vi "Main.vi"() -> ()   [LabVIEW 2020]
uses:
  System.Windows.Forms
  Global_Variable/Global.vi
  Global_Variable/A180648.vi
  <userlib>/_MGI/Menu Building/MenuTypes/MenuStrip/MGI_MenuStrip.lvclass
  <userlib>/_MGI/Menu Building/MenuItemStatusChange/MGI_MenuItemStatusChange.lvclass
  Libraries/S7/S7.lvlib
panel:
  in  "表格控件":string[][](table)
  out "上学状态":string
  in  "Andon":enum32{"未选择", "缺料报警", "质量报警", "故障报警"}(radio)
  out "PLC":bool
  in  "菜单":refnum<k24>(container)
  out "逆向空载":bool
  out "试验计时":u16
  out "产品编号":string
  out "生产数量":i32
  out "合格数量":i32
  out "userStatus":string caption="用户状态"
  out "userName":string caption="用户名"
  out "connectionMode":string caption="联机类型"
  out "产品型号":string
  out "手柄开启力":bool
  out "手柄锁紧力":bool=TRUE
  out "振动NVH":bool
  out "备用试验1":bool
  out "备用试验2":bool
  out "手柄保持力":bool=TRUE caption="管柱保持力"
  out "锁紧/开启":bool
  out "手柄推拉力":bool caption="角度调节力"
  in  "更换产品":refnum<vi>
  out "提示信息":string
  out "错误":bool
  out "时间字符串":string
  out "日期字符串":string
  out "自动":bool
  # "手柄调节机构"
  # "试验项目"
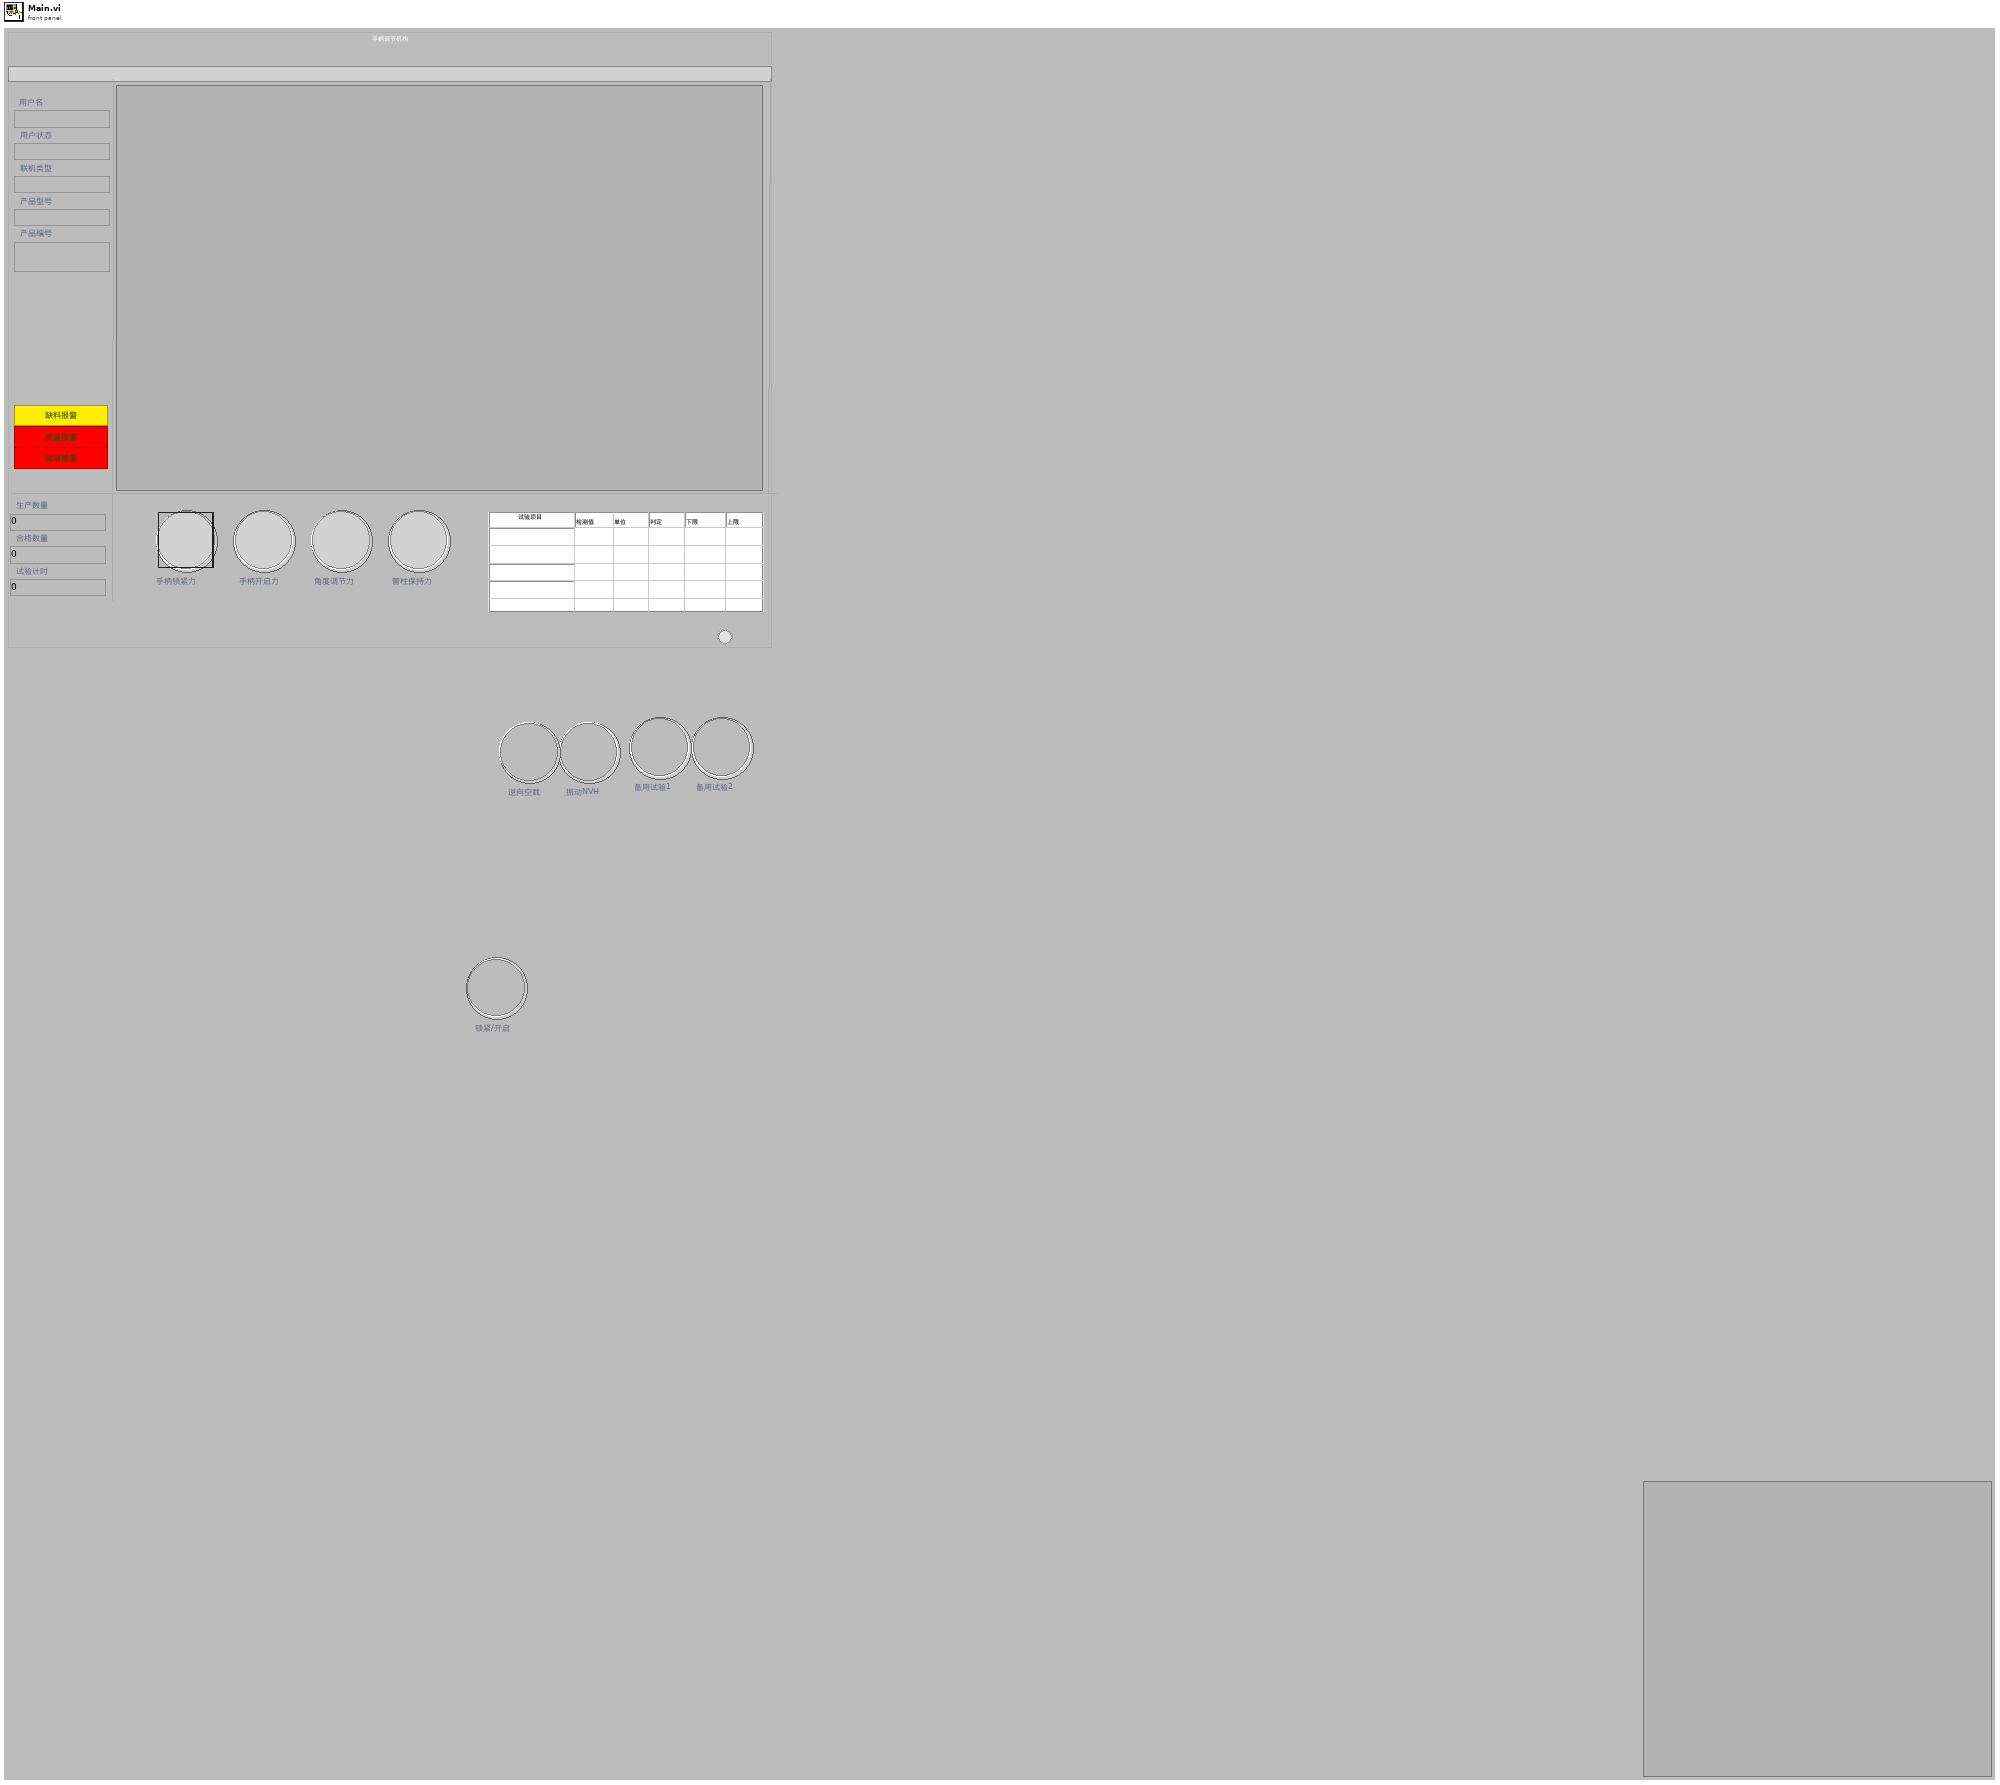
[diagram p1: front panel]
types:
  T1 = typedef "S7.lvlib/Broadcast Events--cluster.ctl" = cluster{"Module Did Init":refnum<user-event>, "Status Updated":refnum<user-event>, "Error Reported":refnum<user-event>, "Module Did Stop":refnum<user-event>, "Update Module Execution Status":refnum<user-event>}
  T2 = enum32{"手柄锁紧力", "手柄开启力", "手柄推拉力", "手柄保持力", "锁紧/松开", "逆向空载", "振动NVH"}
  T3 = enum32{"手柄锁紧力", "手柄开启力", "手柄推拉力", "手柄保持力", "锁紧/开启", "逆向空载", "振动NVH"}
  T4 = enum32{"空载", "功能", "力特性", "电流特性", "传感器特性", "逆向空载", "振动NVH"}
  T5 = enum32{"Invalid", "Standard", "Closed", "Hidden", "Minimized", "Maximized"}
  T6 = cluster{"设备名称":string, "操作人员":string, "设备状态":enum16{"设备离线", "设备正常", "设备缺料", "设备故障", "质量报警"}, "附加信息":string}
  T7 = enum32{"invalid app kind", "Development System", "Run Time System", "Student Edition", "Embedded LabVIEW", "Evaluation", "Custom"}
  T8 = cluster{"操作员编号":string, "操作员姓名":string, "操作员权限":string, "联机模式":enum16{"单机", "追溯"}}
  T9 = cluster{"Core":cluster{"Current VI Reference":refnum<vi>, "Close Panel on Exit?":bool}, "Your Boolean data":bool, "Your string data":string}
  T10 = cluster{"Current VI Reference":refnum<vi>, "Close Panel on Exit?":bool}
  T11 = cluster{"用户编号":string, "用户名":string, "用户密码(密文)":string, "用户权限":string}
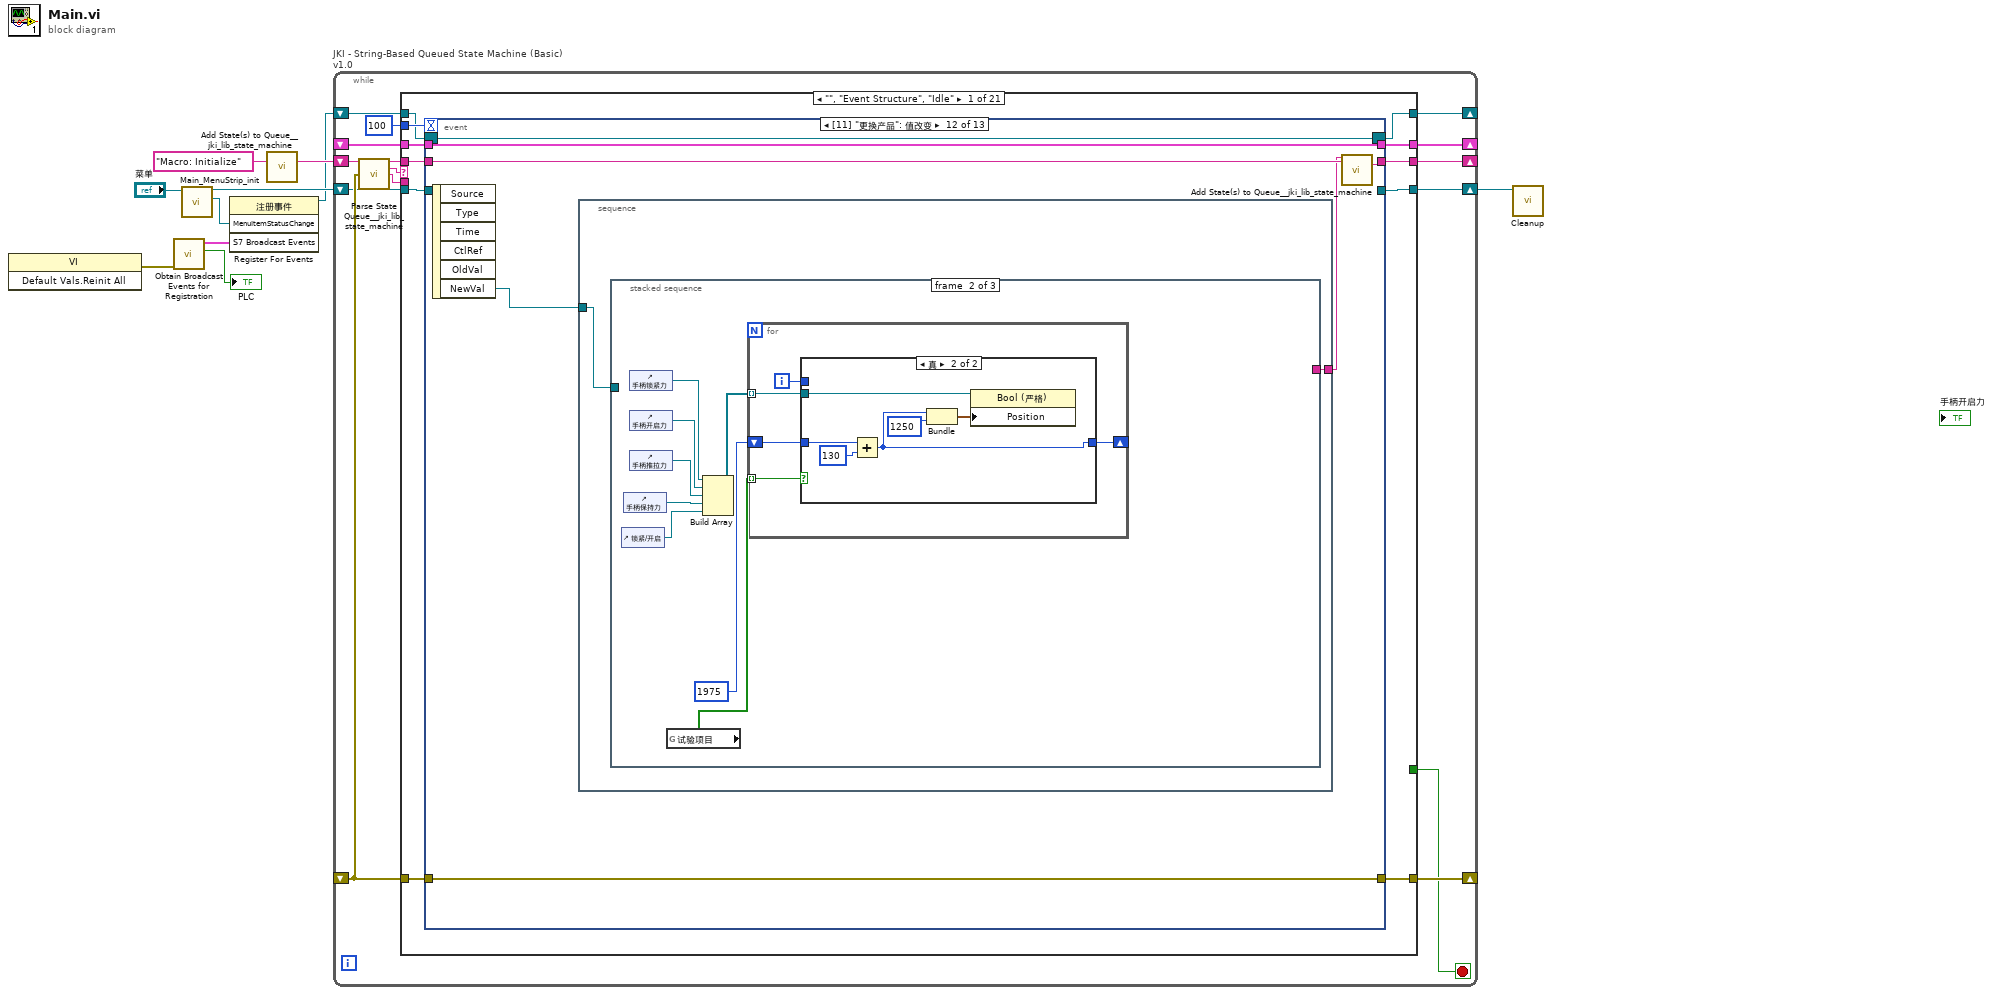
[diagram p0: block diagram]
diagram:
  n1 = invoke class="VI" method="Default Vals.Reinit All"() -> (error out=w3:errorcluster)  [unwired: 3 in, 2 out]
  n2 = call "Obtain Broadcast Events for Registration.vi"("error in (no error)"=w3) -> ("Already running?"=→"PLC":bool, "S7 Broadcast Events"=w5:T1)  [unwired: 8 in, 1 out]
  n3 = call "Main_MenuStrip_init.vi"("MenuStrip"="菜单") -> ("MenuItemStatusChange"=w2:refnum<user-event>, "Menu out"=w7:refnum<class "MGI_MenuStrip.lvclass">)  [unwired: 9 in]
  n4 = register-events(w2, w5) -> (reference out=w1:refnum<event-registration>)  [unwired: 2 in, 1 out]
  n5 = call <vilib>:"Add State(s) to Queue__jki_lib_state_machine.vi"("State(s) in (\"\")"="Macro: Initialize") -> ("States Out"=w10:string)  [unwired: 14 in]
  n6 = while "JKI - String-Based Queued State Machine (Basic) v1.0" {
    shift-right: [w19] -> _
    shift-left: _ -> [w18]
    shift-right: [w21] -> _
    shift-left: _ -> [w16]
    shift-right: [w20] -> _
    shift-left: w10 -> [w22]
    shift-right: [w14] -> w6
    shift-left: w7 -> [w15]
    shift-right: [w12] -> _
    shift-left: w1 -> [w11]
    stop <- w13 stop-if-true
    n7 = call <vilib>:"Parse State Queue__jki_lib_state_machine.vi"("State Queue"=w22, "Error In (no error)"=w16) -> ("Remaining States"=w24:string, "Current State"=w25:string, "Arguments"=w23:string)  [unwired: 11 in]
    n8 = case shown="\"\", \"Event Structure\", \"Idle\"" w25 {
      selector: w25 -> [_ _ w278 _ _ _ _ _ _ _ _ _ _ _ _ _ _ _ _ _ _]
      tunnel: w24 -> [w36 w275 w282 w302 w310 w318 w324 w328 w334 w343 w355 w363 w369 w379 w403 w443 w451 w464 w492 w499 w511]
      tunnel: w23 -> [_ _ _ _ _ _ _ _ _ _ _ _ _ _ _ _ w446 w458 _ _ _]
      tunnel: w18 -> [w34 w272 w280 w293 w307 w316 w321 w329 w337 w340 _ w358 w366 w377 w401 w440 w449 w460 w489 w496 w508]
      tunnel: [w33 w273 w284 w299 errorcluster {"status"=FALSE, "code"=0, "source"=""} ("error out") w315 w322 w326 w332 w341 w352 w359 w367 w376 w399 w441 w447 w461 w490 w497 w509] -> w21
      tunnel: w16 -> [w32 w273 w283 w299 w306 w315 w322 w326 w333 w341 w352 w360 w367 w373 w399 w441 w448 w462 w490 w497 w509]
      tunnel: [w35 w274 w281 w301 w309 w317 w323 w328 w335 w342 w354 w362 w368 w378 w402 w442 w450 w463 w491 w498 w510] -> w20
      tunnel: [w31 w272 w280 w300 w307 w316 w321 w329 w337 w340 w353 w358 w366 w377 w401 w440 w449 w460 w489 w496 w508] -> w19
      tunnel: 100 ("Timeout") -> [w30 _ _ _ _ _ _ _ _ _ _ _ _ _ _ _ _ _ _ _ _]
      tunnel: w15 -> [w29 w271 w277 w290 w304 w314 w320 w327 w336 w339 w346 w357 w365 w375 w400 w439 w445 w457 w488 w494 w501]
      tunnel: [w28 w271 w277 w290 w304 w314 w320 w327 w336 w339 w346 w357 w365 w375 w400 w439 w445 w457 w488 w494 w501] -> w14
      tunnel: [_ _ _ _ _ TRUE _ _ _ _ _ _ _ _ _ _ _ _ _ _ _] -> w13
      tunnel: [w26 w270 w276 w289 w303 w312 w319 w330 w331 w338 w347 w356 w364 w374 w398 w436 w444 w456 w487 w493 w500] -> w12
      tunnel: w11 -> [w27 w270 w276 w289 w303 w312 w319 w330 w331 w338 w347 w356 w364 w374 w398 w436 w444 w456 w487 w493 w500]
      frame "", "Event Structure", "Idle" {
        n9 = event shown="[11] \"更换产品\": 值改变" {
          selector: w27 -> [w38 w63 w84 w90 w156 w163 w170 w177 w191 w200 w207 w216 _]
          dyn-events: [w38 w63 w83 w90 w156 w163 w170 w177 w191 w200 w207 w216 _] -> w26
          timeout: w30 -> [_ _ _ _ _ _ _ _ _ _ _ _ _]
          tunnel: w36 -> [w50 w66 w88 w99 w157 w164 w173 w180 w188 w204 w214 w218 w264]
          tunnel: [w49 w65 w88 w97 w158 w165 w174 w181 w189 w205 w213 w219 w264] -> w35
          tunnel: w34 -> [w48 w67 w89 w98 w160 w168 w175 w182 w190 w206 w211 w221 w265]
          tunnel: [w39 w64 w85 w100 w161 w166 w171 w183 w186 w203 w212 w220 w262] -> w33
          tunnel: w32 -> [w39 w64 w86 w100 w161 w166 w171 w184 w186 w203 w212 w220 w262]
          tunnel: [w48 w67 w89 w98 w160 w168 w175 w182 w190 w206 w211 w221 w265] -> w31
          tunnel: w29 -> [w37 _ w87 w93 w159 w167 w172 w179 w187 _ _ _ w263]
          tunnel: [w37 _ w87 w93 w159 w167 w172 w179 w187 _ _ _ w263] -> w28
          event Timeout {
            n10 = event-data() -> ()  [unwired: 1 in, 1 out]
            n11 = global read "Global.vi" "计时开始"() -> (w41:bool)
            n12 = case shown="真" w41 {
              frame False {
                n13 = global write "Global.vi" "计时复位"(TRUE ("计时复位")) -> ()
              }
              frame True {
                n14 = stacked-sequence {
                  frame #0 {
                    n15 = global read "Global.vi" "计时复位"() -> (w52:bool)
                    n16 = call "已用时间"("Reset"=w52) -> ("Elapsed Time (s)"=→"试验计时":dbl)  [unwired: 11 in, 7 out]
                  }
                  frame #1 {
                    n17 = global write "Global.vi" "计时复位"(FALSE ("计时复位")) -> ()
                  }
                }
              }
            }
            n18 = Format Date/Time String(time format string (%c)="%H:%M ") -> (date/time string=→"时间字符串":string)  [unwired: 2 in]
            n19 = Format Date/Time String(time format string (%c)="%Y年%m月%d日") -> (date/time string=→"日期字符串":string)  [unwired: 2 in]
            n20 = call <vilib>:"Add State(s) to Queue__jki_lib_state_machine.vi"("State(s) in (\"\")"=w50) -> ("States Out"=w49:string)  [unwired: 14 in]
            n21 = global read "Global.vi" "合格数量"() -> (→"合格数量":i32)
            n22 = global read "Global.vi" "生产数量"() -> (→"生产数量":i32)
            n23 = global read "Global.vi" "产品编号"() -> (→"产品编号":string)
          }
          event "手柄锁紧力", "手柄开启力", "手柄推拉力", "手柄保持力", "锁紧/开启", "振动NVH", "逆向空载": Mouse Down {
            w55 = refnum<user-event> refnum items=["手柄锁紧力", "手柄开启力", "手柄推拉力", "手柄保持力", "锁紧/开启", "逆向空载", "振动NVH"] ("试验项_Event")
            n24 = event-data() -> ("CtlRef"=w59:refnum<vi>)  [unwired: 1 in]
            n25 = property class="Bool (严格)"(reference=w59) -> ("Label.Text"=w58:string)  [unwired: 1 in, 2 out]
            n26 = vi-ref "Auto.vi"() -> (w61:refnum<vi>)
            n27 = case shown="\"锁紧/开启\"" w58 {
              tunnel: [T2."手柄锁紧力" ("事件数据") T2."手柄开启力" ("事件数据") T2."手柄推拉力" ("事件数据") T2."手柄保持力" ("事件数据") T3."锁紧/开启" ("事件数据") T4."逆向空载" ("事件数据") T4."振动NVH" ("事件数据")] -> w56
              frame "手柄锁紧力", Default {
              }
              frame "手柄开启力" {
              }
              frame "手柄推拉力" {
              }
              frame "手柄保持力" {
              }
              frame "锁紧/开启" {
              }
              frame "逆向空载" {
              }
              frame "振动NVH" {
              }
            }
            n28 = invoke class="VI" method="Ctrl Val.Get"(reference=w61, "Control Name"="试验项_Event" ("控件名")) -> ("Get Control Value Variant"=w60:variant)  [unwired: 2 in, 3 out]
            n29 = Variant To Data(type=w55, Variant=w60) -> (data=w57:refnum<user-event>)  [unwired: 1 in, 1 out]
            n30 = Generate User Event(user event=w57, event data cluster=w56) -> ()  [unwired: 2 in, 2 out]
            n31 = call <vilib>:"Add State(s) to Queue__jki_lib_state_machine.vi"("State(s) in (\"\")"=w66) -> ("States Out"=w65:string)  [unwired: 14 in]
          }
          event "PLC": Value Change; "PLC": Mouse Down {
            n32 = event-data() -> ()  [unwired: 1 in, 4 out]
            n33 = call "Start Module.vi"("error in (no error)"=w86) -> ("error out"=w79:errorcluster, "Wait for Event Sync?"=w82:bool, "S7 Broadcast Events"=w81:T1, "Module Was Already Running?"=w80:bool)  [unwired: 7 in]
            n34 = local write "PLC"(w80) -> ()
            n35 = register-events(reference=w84, error in=w79, w81) -> (reference out=w83:refnum<event-registration>, error out=w78:errorcluster)  [unwired: 1 in]
            n36 = call "Synchronize Module Events.vi"("error in (no error)"=w78, "Wait for Event Sync?"=w82) -> ("error out"=w75:errorcluster)  [unwired: 9 in]
            n37 = call "Init S7 Link.vi"("error in (no error)"=w75, "超时"=500, "IP"="192.168.0.131") -> ("error out"=w85:errorcluster)  [unwired: 8 in]
          }
          event User Event {
            n38 = event-data() -> ("StatusChange"=w91:refnum<class "MGI_MenuItemStatusChange.lvclass">)  [unwired: 1 in]
            n39 = call <userlib>:"BasicInfo.vi"("MGI_MenuItemStatusChange in"=w91) -> ("Enabled?"=w94:bool, "Checked?"=w95:bool, "Tag"=w96:string)  [unwired: 7 in, 1 out]
            n40 = case shown="\"数据库配置\"" w96 {
              tunnel: w95 -> [_ _ _ _ _ _ _ _ _ _ _ _ _ _ _]
              tunnel: w94 -> [_ _ _ _ _ _ _ _ _ _ _ _ _ _ _]
              tunnel: [_ _ "S7: Stop\nMacro: Exit" _ _ _ _ _ _ _ _ _ _ _ _] -> w92
              frame "假", Default {
              }
              frame "数据库配置" {
                n41 = global read "用户信息.vi" "用户信息"() -> (w102:T8)
                n42 = Unbundle By Name(w102) -> ("操作员权限"=w101:string)
                n43 = case shown="\"系统管理员\"" w101 {
                  frame Default {
                    n44 = One Button Dialog(message="权限不足！" ("消息")) -> ()  [unwired: 1 in, 1 out]
                  }
                  frame "系统管理员" {
                    n45 = vi-ref "数据库配置.vi"() -> (w105:refnum<vi>)
                    n46 = call "CallVI.vi"("VI引用"=w105, "状态"=T5."Standard") -> ()  [unwired: 12 in, 2 out]
                  }
                }
              }
              frame "退出" {
                n47 = global write "Global.vi" "程序关闭"(TRUE ("程序关闭")) -> ()
                n48 = call "Close_Client.vi"() -> ()  [unwired: 12 in]
              }
              frame "手动控制" {
                n49 = global read "用户信息.vi" "用户信息"() -> (w109:T8)
                n50 = Unbundle By Name(w109) -> ("操作员权限"=w108:string)
                n51 = case shown="\"班组长\", \"系统管理员\"" w108 {
                  frame Default {
                    n52 = One Button Dialog(message="权限不足！" ("消息")) -> ()  [unwired: 1 in, 1 out]
                  }
                  frame "班组长", "系统管理员" {
                    n53 = vi-ref "IO.vi"() -> (w112:refnum<vi>)
                    n54 = call "CallVI.vi"("VI引用"=w112, "状态"=T5."Standard") -> ()  [unwired: 12 in, 2 out]
                  }
                }
              }
              frame "半自动控制" {
                n55 = disable-structure shown="启用" {
                  frame Disabled {
                    n56 = shared-variable "我的电脑\\Global.lvlib\\操作者权限"() -> (w113:string)  [unwired: 1 in, 1 out]
                    n57 = case shown="\"班组长\", \"系统管理员\"" w113 {
                      frame Default {
                        n58 = One Button Dialog(message="权限不足！" ("消息")) -> ()  [unwired: 1 in, 1 out]
                      }
                      frame "班组长", "系统管理员" {
                        n59 = call "CallVI.vi"("VI引用"=refnum<vi> refnum, "状态"=T5."Maximized") -> ()  [unwired: 12 in, 2 out]
                      }
                    }
                  }
                  frame Enabled {
                    n60 = One Button Dialog(message="当前设备不具备半自动功能！" ("消息")) -> ()  [unwired: 1 in, 1 out]
                  }
                }
              }
              frame "产品管理" {
                n61 = vi-ref "Config.vi"() -> (w119:refnum<vi>)
                n62 = call "CallVI.vi"("VI引用"=w119, "状态"=T5."Standard") -> ()  [unwired: 12 in, 2 out]
              }
              frame "系统配置" {
                n63 = global read "用户信息.vi" "用户信息"() -> (w121:T8)
                n64 = Unbundle By Name(w121) -> ("操作员权限"=w120:string)
                n65 = case shown="\"班组长\", \"系统管理员\"" w120 {
                  frame Default {
                    n66 = One Button Dialog(message="权限不足！" ("消息")) -> ()  [unwired: 1 in, 1 out]
                  }
                  frame "班组长", "系统管理员" {
                    n67 = vi-ref "Setting.vi"() -> (w124:refnum<vi>)
                    n68 = call "CallVI.vi"("VI引用"=w124, "状态"=T5."Standard") -> ()  [unwired: 12 in, 2 out]
                  }
                }
              }
              frame "用户管理" {
                n69 = global read "用户信息.vi" "用户信息"() -> (w126:T8)
                n70 = Unbundle By Name(w126) -> ("操作员权限"=w125:string)
                n71 = case shown="\"系统管理员\"" w125 {
                  frame Default {
                    n72 = One Button Dialog(message="权限不足！" ("消息")) -> ()  [unwired: 1 in, 1 out]
                  }
                  frame "系统管理员" {
                    n73 = vi-ref "User_manager.vi"() -> (w129:refnum<vi>)
                    n74 = call "CallVI.vi"("VI引用"=w129, "状态"=T5."Standard") -> ()  [unwired: 12 in, 2 out]
                  }
                }
              }
              frame "编码规则" {
                n75 = global read "用户信息.vi" "用户信息"() -> (w131:T8)
                n76 = Unbundle By Name(w131) -> ("操作员权限"=w130:string)
                n77 = case shown="\"班组长\", \"工艺管理员\", \"系统管理员\"" w130 {
                  frame Default {
                    n78 = One Button Dialog(message="权限不足！" ("消息")) -> ()  [unwired: 1 in, 1 out]
                  }
                  frame "班组长", "工艺管理员", "系统管理员" {
                    n79 = vi-ref "编码规则设置.vi"() -> (w134:refnum<vi>)
                    n80 = call "CallVI.vi"("VI引用"=w134, "状态"=T5."Standard") -> ()  [unwired: 12 in, 2 out]
                  }
                }
              }
              frame "易损件管理" {
                n81 = vi-ref "易损件管理.vi"() -> (w136:refnum<vi>)
                n82 = call "CallVI.vi"("VI引用"=w136, "状态"=T5."Standard") -> ()  [unwired: 12 in, 2 out]
              }
              frame "物料批次管理" {
                n83 = vi-ref "批次管理.vi"() -> (w138:refnum<vi>)
                n84 = call "CallVI.vi"("VI引用"=w138, "状态"=T5."Standard") -> ()  [unwired: 12 in, 2 out]
              }
              frame "报表" {
                n85 = call "文件对话框"("start path"=path "D:/report", "prompt"="打开报表", "pattern (all files)"="*.doc;*.docx", "pattern label"="Word 文档") -> ("selected path"=w139:path, "error out"=w140:errorcluster)  [unwired: 8 in, 2 out]
                n86 = case shown="无错误" w140 {
                  selector: w140 -> [w146 w148]
                  tunnel: w139 -> [w147 _]
                  frame No Error {
                    w145 = 1 items=["Normal", "Maximize", "Minimize"] ("cpubbs_WindowState")
                    n87 = call "Open_Word.vi"("File Path"=w147, "cpubbs_WindowState"=w145, "错误输入（无错误）"=w146) -> ()  [unwired: 12 in, 1 out]
                  }
                  frame Error {
                    n88 = call <vilib>:"Clear Errors.vi"("error in (no error)"=w148) -> ()  [unwired: 5 in, 2 out]
                  }
                }
              }
              frame "报警信息" {
                n89 = vi-ref "报警信息.vi"() -> (w150:refnum<vi>)
                n90 = call "CallVI.vi"("VI引用"=w150, "状态"=T5."Standard") -> ()  [unwired: 12 in, 2 out]
              }
              frame "关于" {
                n91 = vi-ref "About.vi"() -> (w152:refnum<vi>)
                n92 = call "CallVI.vi"("VI引用"=w152, "状态"=T5."Standard") -> ()  [unwired: 12 in, 2 out]
              }
              frame "操作演示" {
                n93 = call <vilib>:"Application Directory.vi"() -> ("Application Directory"=w155:path)
                n94 = Build Path(base path=w155, name or relative path="操作演示" ("名称或相对路径")) -> (appended path=w154:path)
                n95 = call "自动播放ppt.vi"("路径"=w154) -> ()  [unwired: 10 in, 1 out]
              }
            }
            n96 = call <vilib>:"Add State(s) to Queue__jki_lib_state_machine.vi"("State(s) in (\"\")"=w99, "State(s) at Back (\"\")"=w92) -> ("States Out"=w97:string)  [unwired: 13 in]
          }
          event User Event {
            n97 = event-data() -> ("Init?"=w162:bool)  [unwired: 1 in, 1 out]
            n98 = local write "PLC"(w162) -> ()
            n99 = call <vilib>:"Add State(s) to Queue__jki_lib_state_machine.vi"("State(s) in (\"\")"=w157) -> ("States Out"=w158:string)  [unwired: 14 in]
          }
          event User Event {
            n100 = event-data() -> ("Running?"=w169:bool)  [unwired: 1 in]
            n101 = local write "PLC"(w169) -> ()
            n102 = call <vilib>:"Add State(s) to Queue__jki_lib_state_machine.vi"("State(s) in (\"\")"=w164) -> ("States Out"=w165:string)  [unwired: 14 in]
          }
          event User Event {
            n103 = event-data() -> ()  [unwired: 1 in, 7 out]
            n104 = local write "PLC"(FALSE ("PLC")) -> ()
            n105 = call <vilib>:"Add State(s) to Queue__jki_lib_state_machine.vi"("State(s) in (\"\")"=w173) -> ("States Out"=w174:string)  [unwired: 14 in]
          }
          event User Event {
            n106 = event-data() -> ("Error"=w185:errorcluster)  [unwired: 1 in]
            n107 = Merge Errors(w185, w184) -> (w183:errorcluster)
            n108 = call <vilib>:"Add State(s) to Queue__jki_lib_state_machine.vi"("State(s) in Front (\"\")"="S7: Initialize\nIdle", "State(s) in (\"\")"=w180) -> ("States Out"=w181:string)  [unwired: 13 in]
          }
          event "自动": Mouse Down {
            n109 = event-data() -> ()  [unwired: 1 in, 1 out]
            n110 = disable-structure shown="启用" {
              frame Disabled {
                n111 = local read "自动"() -> (w192:bool)
                n112 = case shown="假" w192 {
                  frame False {
                    n113 = call "设备状态.vi"() -> ("Status_Read"=w193:i16)  [unwired: 11 in]
                    n114 = case shown="5" w193 {
                      frame 0, Default {
                        n115 = One Button Dialog(message="请复位！" ("消息")) -> ()  [unwired: 1 in, 1 out]
                      }
                      frame 5 {
                      }
                    }
                  }
                  frame True {
                    n116 = Two Button Dialog(message="确定要退出自动？" ("消息")) -> (T button?=w195:bool)  [unwired: 2 in]
                    n117 = case shown="真" w195 {
                      frame False {
                      }
                      frame True {
                        n118 = vi-ref "Auto.vi"() -> (w199:refnum<vi>)